vi "HFRR ADV v039.vi"() -> ()   [LabVIEW 2025] (continued)
                  tunnel: [w3880] -> w3851
                  n3077 = call-dynamic "Set Report Tab Width.vi"("report in"=w3883, "error in (no error)"=w3881) -> ("report out"=w3882:refnum<class "NI_report.lvclass">, "error out"=w3880:errorcluster)  [unwired: 12 in]
                }
                n3078 = control-ref of="Tab Control 9"() -> (w3847:refnum<vi>)
                n3079 = call-dynamic "Append Control Image to Report.vi"("report in"=w3852, "alignment (default)"=HTML_Report_Image_Alignment."ABSMIDDLE", "ctrl reference"=w3847, "error in (no error)"=w3851) -> ("report out"=w3846:refnum<class "NI_report.lvclass">, "error out"=w3845:errorcluster)  [unwired: 8 in, 2 out]
                n3080 = for {
                  N: 3 -> [_]
                  tunnel: [w3879] -> w3830
                  tunnel: [w3878] -> w3829
                  tunnel: w3846 -> [w3877]
                  tunnel: w3845 -> [w3876]
                  n3081 = call-dynamic "New Report Line.vi"("report in"=w3877, "error in (no error)"=w3876) -> ("report out"=w3879:refnum<class "NI_report.lvclass">, "error out"=w3878:errorcluster)  [unwired: 12 in]
                }
                n3082 = for {
                  N: 100 -> [_]
                  tunnel: w3830 -> [w3875]
                  tunnel: w3829 -> [w3873]
                  tunnel: [w3874] -> w3826
                  tunnel: [w3872] -> w3824
                  n3083 = call-dynamic "Set Report Tab Width.vi"("report in"=w3875, "error in (no error)"=w3873) -> ("report out"=w3874:refnum<class "NI_report.lvclass">, "error out"=w3872:errorcluster)  [unwired: 12 in]
                }
                n3084 = String To Path(string="C:\\LAB-IQ\\im\\Temp_resized.jpg") -> (path=w3816:path)
                n3085 = call-poly <vilib>:"Append Image to Report.vi"("report in"=w3826, "path or URL of image"=w3816, "error in (no error)"=w3824) -> ("report out"=w3825:refnum<class "NI_report.lvclass">, "error out"=w3823:errorcluster)  [unwired: 9 in, 2 out]
                n3086 = call-poly <vilib>:"Open HTML Report in Browser.vi"("report in"=w3825, "error in (no error)"=w3823) -> ("report out"=w3860:refnum<class "NI_report.lvclass">, "error out"=w3859:errorcluster)  [unwired: 11 in, 1 out]
                n3087 = call-dynamic "Dispose Report.vi"("report in"=w3860, "error in (no error)"=w3859) -> ()  [unwired: 13 in, 1 out]
              }
              frame #2 {
              }
              frame #3 {
                n3088 = disable-structure shown="Disabled" {
                  frame Disabled {
                    n3089 = local read "String 10"() -> (w3900:string)
                    n3090 = Concatenate Strings("C:\\LAB-IQ-NXT\\Data\\" ("string"), w3900, ".jpg" ("string")) -> (w3898:string)
                    n3091 = String To Path(string=w3898) -> (path=w3897:path)
                    n3092 = Delete(path (use dialog)=w3897) -> ()  [unwired: 4 in, 3 out]
                  }
                  frame Enabled {
                  }
                }
                n3093 = local write "Print 2"(FALSE ("Print")) -> ()
              }
            }
          }
        }
      }
    }
    n3094 = Wait (ms)(milliseconds to wait=u32 50) -> ()  [unwired: 1 out]
    n3095 = Wait (ms)(milliseconds to wait=u32 50) -> ()  [unwired: 1 out]
    n3096 = local read "Quit"() -> (w2242:bool)
  }
  n3097 = VISA Close(VISA resource name=w41, error in (no error)=w40) -> ()  [unwired: 1 out]
  n3098 = while {
    stop <- w4051 stop-if-true
    n3099 = local read "Auto Start Test"() -> (w4049:bool)
    n3100 = local read "RUN"() -> (w4048:bool)
    n3101 = Wait (ms)(milliseconds to wait=u32 1000) -> ()  [unwired: 1 out]
    n3102 = Or(x=w4048, y=w4049) -> (x .or. y?=w4047:bool)
    n3103 = case shown="True" w4047 {
      frame False {
      }
      frame True {
        n3104 = local read "LVDT STROKE Actual"() -> (w4052:dbl)
        n3105 = In Range and Coerce(upper limit=1.2, x=w4052, lower limit=0.6) -> (In Range?=w4055:bool)  [unwired: 1 out]
        n3106 = call-poly <vilib>:"Random Number (Range).vi"("lower bound (0)"=0.998 ("upper bound (100)"), "upper bound (100)"=1.003) -> ("number"=w4053:dbl)  [unwired: 9 in]
        n3107 = case shown="True" w4055 {
          tunnel: [w4060 w4061] -> w4054
          tunnel: w4053 -> [_ w4061]
          tunnel: w4052 -> [w4060 _]
          frame False {
          }
          frame True {
          }
        }
        "LVDT STROKE DISPLAY" <- w4054
      }
    }
    n3108 = local read "Quit"() -> (w4051:bool)
  }
  n3109 = while {
    tunnel: [w4078] -> w49
    shift-right: [w4071] -> _
    shift-left: 0.0 -> [w4074]
    shift-right: [w4070] -> _
    shift-left: 0.0 -> [w4073]
    shift-right: [w4069] -> _
    shift-left: 100.0 ("vc_cmd") -> [w4072]
    stop <- w4078 stop-if-true
    # "PID LOGIC"
    n3110 = local read "run test Calibration"() -> (w4066:bool)
    n3111 = local read "RUN"() -> (w4076:bool)
    n3112 = local read "Auto Start Temp"() -> (w4067:bool)
    n3113 = local read "Auto Start Test"() -> (w4075:bool)
    n3114 = local read "START TEMP"() -> (w4065:bool)
    n3115 = And(x=w4067, y=w4075) -> (x .and. y?=w4068:bool)
    n3116 = Or(x=w4076, y=w4068) -> (x .or. y?=w4077:bool)
    n3117 = And(x=w4077, y=w4065) -> (x .and. y?=w4064:bool)
    n3118 = And(x=w4066, y=w4065) -> (x .and. y?=w4063:bool)
    n3119 = Or(x=w4063, y=w4064) -> (x .or. y?=w4062:bool)
    n3120 = Wait (ms)(milliseconds to wait="milliseconds to wait") -> ()  [unwired: 1 out]
    n3121 = case shown="True" w4062 {
      tunnel: [400.0 ("out_vc_cmd") w4097] -> w4069
      tunnel: [w4081 w4099] -> w4070
      tunnel: [w4081 w4098] -> w4071
      tunnel: w4074 -> [_ w4088]
      tunnel: w4073 -> [_ w4087]
      tunnel: w4072 -> [_ w4086]
      tunnel: w4066 -> [_ w4082]
      frame False {
        w4081 = 0.0 ("error_out")
      }
      frame True {
        n3122 = case shown="True" w4082 {
          tunnel: [w4106 1.0] -> w4084
          frame False {
            n3123 = local read "Set Strk"() -> (w4105:dbl)
            n3124 = Add(x=w4105, y="Add up Stroke") -> (x+y=w4106:dbl)
          }
          frame True {
          }
        }
        n3125 = local read "LVDT STROKE"() -> (w4083:dbl)
        n3126 = formula code="// Zero-Hardcode Explicit Positional-Form PID Engine\n// Inputs: target_stroke, measured_stroke, dt, prev_error, integral_accumulator_in, prev_vc_cmd\n//         kp, ki, kd, max_step_change, max_amplitude, min_amplitude, startup_cmd\n// Outputs: vc_cmd, error_out, out_error, integral_accumulator_out, out_vc_cmd\n\n// 1. Calculate Tracking Error\nfloat current_error = target_stroke - measured_stroke;\nerror_out = current_error;\n\n// 2. Compute Proportional Term\nfloat p_term = kp * current_error;\n\n// 3. Compute Derivative Term\nfloat d_term = 0.0;\nif (dt > 0.0) {\n    d_term = kd * ((current_error - prev_error) / dt);\n}\n\n// 4. Update and Accumulate Integral Term\nfloat current_integral = integral_accumulator_in + (current_error * dt);\nfloat i_term = ki * current_integral;\n\n// 5. Calculate Ideal Target Command (Anchored by startup baseline)\nfloat ideal_command = startup_cmd + p_term + i_term + d_term;\n\n// 6. Apply Loop Rate Limiting FIRST \n// (Forces the command to climb gradually from prev_vc_cmd instead of jumping straight to max)\nfloat raw_adjustment = ideal_command - prev_vc_cmd;\n\nif (raw_adjustment > max_step_change) {\n    raw_adjustment = max_step_change;\n} else if (raw_adjustment < -max_step_change) {\n    raw_adjustment = -max_step_change;\n}\n\nfloat next_vc_cmd = prev_vc_cmd + raw_adjustment;\n\n// 7. Anti-Windup Protection & Final Output Safety Safeguard Clamping\n// (Back-calculating based on what we are ACTUALLY outputting)\nif (next_vc_cmd > max_amplitude) {\n    float excess = next_vc_cmd - max_amplitude;\n    if (ki > 0.0) {\n        current_integral -= excess / ki;\n    }\n    next_vc_cmd = max_amplitude;\n} else if (next_vc_cmd < min_amplitude) {\n    float excess = next_vc_cmd - min_amplitude;\n    if (ki > 0.0) {\n        current_integral -= excess / ki;\n    }\n    next_vc_cmd = min_amplitude;\n}\n\n// 8. Map to Shift Registers for memory persistence\nvc_cmd = next_vc_cmd;\nout_error = current_error;                   \nintegral_accumulator_out = current_integral;  \nout_vc_cmd = next_vc_cmd;"("target_stroke"=w4084, "measured_stroke"=w4083, "dt"="dt", "integral_accumulator_in"=w4087, "prev_error"=w4088, "prev_vc_cmd"=w4086, "kp"="kp", "ki"="ki", "kd"="kd", "max_step_change"="max_step_change", "max_amplitude"="max_amplitude", "min_amplitude"="min_amplitude", "startup_cmd"="startup_cmd") -> ("vc_cmd"=w4103:dbl, "out_error"=w4098:dbl, "integral_accumulator_out"=w4099:dbl, "out_vc_cmd"=w4097:dbl)  [unwired: 1 out]
        "output Vpp" <- w4103
        n3127 = Number To Fractional String(number=w4103, precision (6)=i16 1) -> (F-format string=w4101:string)  [unwired: 2 in]
        n3128 = Concatenate Strings("DAC;" ("string"), w4101) -> (w4085:string)
        n3129 = local write "Due Write"(w4085) -> ()
        "prev_error" <- w4088
        "integral_accumulator_in" <- w4087
        "prev_vc_cmd" <- w4086
      }
    }
    n3130 = local read "Quit"() -> (w4078:bool)
  }
  n3131 = Or(x=w45, y=w44) -> (x .or. y?=w46:bool)
  n3132 = Or(x=w42, y=w46) -> (x .or. y?=w51:bool)
  n3133 = control-ref of="new picture"() -> ()  [unwired: 1 out]
  n3134 = Or(x=w54, y=w51) -> (x .or. y?=w48:bool)
  n3135 = Or(x=w48, y=w49) -> (x .or. y?=w43:bool)
  n3136 = while {
    tunnel: [w4108] -> w53
    i -> [w4115]
    stop <- w4108 stop-if-true
    n3137 = local read "Quit"() -> (w4108:bool)
    n3138 = Equal To 0?(x=w4115) -> (x = 0?=w4113:bool)
    n3139 = call "Elapsed Time3"("Time Target (s)"=45.0, "Auto Reset"=TRUE) -> ("Time has Elapsed"=w4112:bool)  [unwired: 10 in, 7 out]
    n3140 = Wait (ms)(milliseconds to wait=u32 50) -> ()  [unwired: 1 out]
    n3141 = Or(x=w4112, y=w4113) -> (x .or. y?=w4114:bool)
    n3142 = case shown="True" w4114 {
      frame False {
      }
      frame True {
        n3143 = call <vilib>:"System Exec.vi"("run minimized? (F)"=TRUE, "error in (no error)"="error in (no error)", "command line"="powercfg.exe -change -monitor-timeout-ac 0") -> ("error out"=w4126:errorcluster)  [unwired: 5 in, 3 out]
        n3144 = call <vilib>:"System Exec.vi"("run minimized? (F)"=TRUE, "error in (no error)"=w4126, "command line"="powercfg.exe -change -disk-timeout-ac 0") -> ("error out"=w4125:errorcluster)  [unwired: 5 in, 3 out]
        n3145 = call <vilib>:"System Exec.vi"("run minimized? (F)"=TRUE, "error in (no error)"=w4125, "command line"="powercfg.exe -change -standby-timeout-ac 0") -> ("error out"=w4124:errorcluster)  [unwired: 5 in, 3 out]
        n3146 = call <vilib>:"System Exec.vi"("run minimized? (F)"=TRUE, "error in (no error)"=w4124, "command line"="powercfg.exe -change -hibernate-timeout-ac 0") -> ("error out"=w4123:errorcluster)  [unwired: 5 in, 3 out]
        n3147 = call <vilib>:"Simple Error Handler.vi"("error in (no error)"=w4123) -> ("error out"=w4129:errorcluster)  [unwired: 4 in, 4 out]
        n3148 = call <vilib>:"Clear Errors.vi"("error in (no error)"=w4129) -> ("error out"=→"error out":errorcluster)  [unwired: 5 in, 1 out]
      }
    }
  }
  n3149 = Compound Arithmetic op=OR(w56, w43, w53) -> (w55:bool)
  n3150 = flat-sequence {
    tunnel: w55 -> [_]
    tunnel: [w4131] -> w25
    tunnel: w25 -> [_]
    frame #0 {
      n3151 = call "CLOSE CONNECTION.vi"() -> ("error out"=w4131:errorcluster)  [unwired: 11 in]
    }
    frame #1 {
      n3152 = Quit LabVIEW(quit? (T)=TRUE) -> ()
      n3153 = local write "Quit"(FALSE ("EXIT")) -> ()
    }
  }
  n3154 = property on="Heater Button" class="Bool (strict)"("Visible"=TRUE) -> ()  [unwired: 2 in, 2 out]
  n3155 = while {
    tunnel: [w4138] -> _
    i -> [w4138]
    stop <- w4134 stop-if-true
    # "Langauage selection"
    n3156 = Equal?(x="Lan flag", y=22.0) -> ()  [unwired: 1 out]
    n3157 = disable-structure shown="Disabled" {
      frame Disabled {
        n3158 = stacked-sequence {
          frame #0 {
            n3159 = case shown="\"Russian\"" "Language Selection" {
              tunnel: [0 1] -> w4140
              frame "English", Default {
              }
              frame "Russian" {
              }
            }
            n3160 = for {
              N: 130 -> [_]
              tunnel: "Table" -> [w4149]
              tunnel: w4140 -> [w4148]
              i -> [w4147]
              n3161 = Index Array(array=w4149, index (row)=w4147, index (col)=w4148) -> (element=w4146:string)
              n3162 = case shown="1" w4147 {
                tunnel: w4146 -> [w4150 w4151 _ w4152 w4153 w4154 w4155 w4156 w4157 w4158 w4159 w4160 w4161 w4162 w4163 w4164 w4165 w4166 w4167 w4168 w4169 w4170 w4171 w4172 w4173 w4174 w4175 w4176 w4177 _ _ w4178 w4179 w4180 w4181 w4182 w4183 w4192 w4199 w4206 w4213 w4217 w4220 w4223 w4225 w4227 w4228 w4229 w4230 w4231 w4232 w4233 w4234 w4235 w4236 w4237 w4238 w4239 w4240 w4241 w4242 w4243 w4244 w4245 w4246 w4247 w4248 w4249 w4250 w4251 w4252 w4253 w4254 w4255 w4256 w4257 w4258 w4259 w4260 w4261 w4262 w4263 w4264 w4265 w4266 w4267 w4268 w4269 w4270 w4271 w4272 w4273 w4274 w4275 w4276 w4277 w4278 w4279 w4280 w4281 w4282 w4283 w4284 w4285 w4286 _ w4287 w4288 w4289 w4290 w4291 w4292 w4293 w4294 w4295 w4296 w4297 w4298 w4299 _ w4300 w4301 w4302 w4303 w4304 w4305 _]
                frame 0 {
                  n3163 = local write "S"(w4150) -> ()
                }
                frame 1 {
                  n3164 = local write "S 2"(w4151) -> ()
                }
                frame 2 {
                }
                frame 3 {
                  n3165 = local write "S 4"(w4152) -> ()
                }
                frame 4 {
                  n3166 = property on="FILE" class="Str"("Caption.Text"=w4153) -> ()  [unwired: 2 in, 2 out]
                }
                frame 5 {
                  n3167 = property on="Fuel Discription :" class="Str"("Caption.Text"=w4154) -> ()  [unwired: 2 in, 2 out]
                }
                frame 6 {
                  n3168 = property on="Remarks :" class="Str"("Caption.Text"=w4155) -> ()  [unwired: 2 in, 2 out]
                }
                frame 7 {
                  n3169 = property on="Save & Continue" class="Bool (strict)"("Boolean Text.Text"=w4156) -> ()  [unwired: 2 in, 2 out]
                }
                frame 8 {
                }
                frame 9 {
                  n3170 = property on="Set Hz" class="DigNum (strict)"("Caption.Text"=w4158) -> ()  [unwired: 2 in, 2 out]
                }
                frame 10 {
                }
                frame 11 {
                  n3171 = property on="NORMAL LOAD" class="DigNum (strict)"("Caption.Text"=w4160) -> ()  [unwired: 2 in, 2 out]
                }
                frame 12 {
                }
                frame 13 {
                  n3172 = property on="Set Temp" class="DigNum (strict)"("Caption.Text"=w4162) -> ()  [unwired: 2 in, 2 out]
                }
                frame 14 {
                  n3173 = local write "S 15"(w4163) -> ()
                }
                frame 15 {
                  n3174 = property on="Set Rh" class="DigNum (strict)"("Caption.Text"=w4164) -> ()  [unwired: 2 in, 2 out]
                }
                frame 16 {
                }
                frame 17 {
                  n3175 = local write "S 18"(w4166) -> ()
                }
                frame 18 {
                  "String 17" <- w4167
                }
                frame 19 {
                  n3176 = property on="test time" class="DigNum (strict)"("Caption.Text"=w4168) -> ()  [unwired: 2 in, 2 out]
                }
                frame 20 {
                  "String 18" <- w4169
                  "String 22" <- w4169
                }
                frame 21 {
                  n3177 = property on="Elapsed time" class="DigNum (strict)"("Caption.Text"=w4170) -> ()  [unwired: 2 in, 2 out]
                }
                frame 22 {
                  n3178 = property on="Samplingtime 2" class="DigNum (strict)"("Caption.Text"=w4171) -> ()  [unwired: 2 in, 2 out]
                }
                frame 23 {
                  "String 21" <- w4172
                }
                frame 24 {
                  n3179 = property on="Countdown" class="DigNum (strict)"("Caption.Text"=w4173) -> ()  [unwired: 2 in, 2 out]
                }
                frame 25 {
                  n3180 = property on="Countdown 2" class="DigNum (strict)"("Caption.Text"=w4174) -> ()  [unwired: 2 in, 2 out]
                }
                frame 26 {
                  n3181 = property on="Engage" class="Bool (strict)"("Boolean Text.Text"=w4175) -> ()  [unwired: 2 in, 2 out]
                }
                frame 27 {
                  n3182 = property on="Boolean  4" class="Bool (strict)"("Boolean Text.Text"=w4176) -> ()  [unwired: 2 in, 2 out]
                }
                frame 28 {
                  n3183 = property on="Test \nStatus" class="Bool (strict)"("Boolean Text.Text"=w4177) -> ()  [unwired: 2 in, 2 out]
                }
                frame 29 {
                }
                frame 30 {
                }
                frame 31 {
                }
                frame 32 {
                  n3184 = property on="RSTCOF" class="Bool"("Boolean Text.Text"=w4179) -> ()  [unwired: 2 in, 2 out]
                  n3185 = property on="RST FF" class="Bool"("Boolean Text.Text"=w4179) -> ()  [unwired: 2 in, 2 out]
                  n3186 = property on="RST TEMP" class="Bool"("Boolean Text.Text"=w4179) -> ()  [unwired: 2 in, 2 out]
                  n3187 = property on="RSTV1 3" class="Bool"("Boolean Text.Text"=w4179) -> ()  [unwired: 2 in, 2 out]
                  n3188 = property on="rstv2" class="Bool"("Boolean Text.Text"=w4179) -> ()  [unwired: 2 in, 2 out]
                  n3189 = property on="RSTV1 2" class="Bool"("Boolean Text.Text"=w4179) -> ()  [unwired: 2 in, 2 out]
                  n3190 = property on="RST CP" class="Bool"("Boolean Text.Text"=w4179) -> ()  [unwired: 2 in, 2 out]
                }
                frame 33 {
                  "S 61" <- w4180
                }
                frame 34 {
                  "String 23" <- w4181
                }
                frame 35 {
                  n3191 = property on="Rh Before" class="DigNum (strict)"("Caption.Text"=w4182) -> ()  [unwired: 2 in, 2 out]
                }
                frame 36 {
                  n3192 = Match Pattern(string=w4183, regular expression=",") -> (before substring=→"bs":string, after substring=→"as":string)  [unwired: 1 in, 2 out]
                  n3193 = property on="Rh After" class="DigNum (strict)"("Caption.Text"=w4183) -> ()  [unwired: 2 in, 2 out]
                }
                frame 37 {
                  n3194 = Match Pattern(string=w4192, regular expression=",") -> (before substring=w4191:string, after substring=w4190:string)  [unwired: 1 in, 2 out]
                  "bs" <- w4191
                  "as" <- w4190
                  n3195 = Concatenate Strings(w4191, w4190) -> (w4187:string)
                  n3196 = property on="Humidity before test 2" class="DigNum (strict)"("Caption.Text"=w4187) -> ()  [unwired: 2 in, 2 out]
                  n3197 = Concatenate Strings(w4187, "=" ("string")) -> (w4188:string)
                  n3198 = local write "S 38"(w4188) -> ()
                }
                frame 38 {
                  n3199 = Match Pattern(string=w4199, regular expression=",") -> (before substring=w4198:string, after substring=w4197:string)  [unwired: 1 in, 2 out]
                  "bs" <- w4198
                  "as" <- w4197
                  n3200 = Concatenate Strings(w4198, w4197) -> (w4194:string)
                  n3201 = property on="Humidity after test 2" class="DigNum (strict)"("Caption.Text"=w4194) -> ()  [unwired: 2 in, 2 out]
                  n3202 = Concatenate Strings(w4194, "=" ("string")) -> (w4196:string)
                  n3203 = local write "S 39"(w4196) -> ()
                }
                frame 39 {
                  n3204 = Match Pattern(string=w4206, regular expression=",") -> (before substring=w4205:string, after substring=w4204:string)  [unwired: 1 in, 2 out]
                  "bs" <- w4205
                  "as" <- w4204
                  n3205 = Concatenate Strings(w4205, w4204) -> (w4201:string)
                  n3206 = property on="Temperature before test 2" class="DigNum (strict)"("Caption.Text"=w4201) -> ()  [unwired: 2 in, 2 out]
                  n3207 = Concatenate Strings(w4201, "=" ("string")) -> (→"String 34":string)
                }
                frame 40 {
                  n3208 = Match Pattern(string=w4213, regular expression=",") -> (before substring=w4212:string, after substring=w4211:string)  [unwired: 1 in, 2 out]
                  "bs" <- w4212
                  "as" <- w4211
                  n3209 = Concatenate Strings(w4212, w4211) -> (w4208:string)
                  n3210 = property on="Temperature after test 2" class="DigNum (strict)"("Caption.Text"=w4208) -> ()  [unwired: 2 in, 2 out]
                  n3211 = Concatenate Strings(w4208, "=" ("string")) -> (→"String 35":string)
                  n3212 = property on="Temperature after test" class="DigNum (strict)"("Caption.Text"=w4208) -> ()  [unwired: 2 in, 2 out]
                }
                frame 41 {
                  n3213 = property on="AVP 2" class="DigNum (strict)"("Caption.Text"=w4217) -> ()  [unwired: 2 in, 2 out]
                  n3214 = Concatenate Strings(w4217, "=" ("string")) -> (→"String 36":string)
                }
                frame 42 {
                  n3215 = property on="MWSD 2" class="DigNum (strict)"("Caption.Text"=w4220) -> ()  [unwired: 2 in, 2 out]
                  n3216 = Concatenate Strings(w4220, "=" ("string")) -> (→"String 37":string)
                }
                frame 43 {
                  n3217 = property on="HCF 2" class="DigNum (strict)"("Caption.Text"=w4223) -> ()  [unwired: 2 in, 2 out]
                  n3218 = Concatenate Strings(w4223, "=" ("string")) -> (→"String 38":string)
                }
                frame 44 {
                  n3219 = Concatenate Strings(w4225, "=" ("string")) -> (→"String 39":string)
                  n3220 = property on="WS1.4 2" class="DigNum (strict)"("Caption.Text"=w4225) -> ()  [unwired: 2 in, 2 out]
                }
                frame 45 {
                }
                frame 46 {
                  n3221 = local write "S 47"(w4228) -> ()
                }
                frame 47 {
                  n3222 = local write "S 48"(w4229) -> ()
                }
                frame 48 {
                  n3223 = local write "S 49"(w4230) -> ()
                }
                frame 49 {
                  n3224 = local write "S 50"(w4231) -> ()
                }
                frame 50 {
                  n3225 = local write "S 51"(w4232) -> ()
                }
                frame 51 {
                  n3226 = local write "S 52"(w4233) -> ()
                }
                frame 52 {
                  n3227 = local write "S 53"(w4234) -> ()
                }
                frame 53 {
                  n3228 = local write "S 54"(w4235) -> ()
                }
                frame 54 {
                  n3229 = local write "S 55"(w4236) -> ()
                }
                frame 55 {
                  n3230 = local write "S 56"(w4237) -> ()
                }
                frame 56 {
                  n3231 = local write "S 57"(w4238) -> ()
                }
                frame 57 {
                  n3232 = local write "S 58"(w4239) -> ()
                }
                frame 58 {
                  n3233 = local write "S 59"(w4240) -> ()
                }
                frame 59 {
                  n3234 = local write "S 60"(w4241) -> ()
                }
                frame 60 {
                  n3235 = local write "S 62"(w4242) -> ()
                }
                frame 61 {
                  n3236 = local write "S 63"(w4243) -> ()
                }
                frame 62 {
                  n3237 = local write "S 64"(w4244) -> ()
                }
                frame 63 {
                  n3238 = local write "S 65"(w4245) -> ()
                }
                frame 64 {
                  n3239 = local write "S 66"(w4246) -> ()
                }
                frame 65 {
                  n3240 = local write "S 67"(w4247) -> ()
                }
                frame 66 {
                  n3241 = local write "S 68"(w4248) -> ()
                }
                frame 67 {
                  n3242 = local write "S 69"(w4249) -> ()
                }
                frame 68 {
                  n3243 = local write "S 70"(w4250) -> ()
                }
                frame 69 {
                  n3244 = local write "S 71"(w4251) -> ()
                }
                frame 70 {
                  n3245 = local write "S 72"(w4252) -> ()
                }
                frame 71 {
                  n3246 = local write "S 73"(w4253) -> ()
                }
                frame 72 {
                  n3247 = local write "S 74"(w4254) -> ()
                }
                frame 73 {
                  n3248 = local write "S 75"(w4255) -> ()
                }
                frame 74 {
                  n3249 = local write "S 76"(w4256) -> ()
                }
                frame 75 {
                  n3250 = local write "S 77"(w4257) -> ()
                }
                frame 76 {
                  n3251 = local write "S 78"(w4258) -> ()
                }
                frame 77 {
                  n3252 = local write "S 79"(w4259) -> ()
                }
                frame 79 {
                  n3253 = property on="Sample Temperature ( °C )" class="XYGraph (strict)"("Y Scale.Name Label.Text"=w4260) -> ()  [unwired: 2 in, 2 out]
                }
                frame 80 {
                  n3254 = local write "S 81"(w4261) -> ()
                  n3255 = property on="Humidity ( %RH )" class="XYGraph (strict)"("Y Scale.Name Label.Text"=w4261) -> ()  [unwired: 2 in, 2 out]
                }
                frame 78 {
                  n3256 = property on="Air Temperature  ( °C )" class="XYGraph (strict)"("X Scale.Name Label.Text"=w4262) -> ()  [unwired: 2 in, 2 out]
                  n3257 = property on="Humidity ( %RH )" class="XYGraph (strict)"("X Scale.Name Label.Text"=w4262) -> ()  [unwired: 2 in, 2 out]
                  n3258 = property on="Sample Temperature ( °C )" class="XYGraph (strict)"("X Scale.Name Label.Text"=w4262) -> ()  [unwired: 2 in, 2 out]
                  n3259 = property on="Coefficient Of Friction" class="XYGraph (strict)"("X Scale.Name Label.Text"=w4262) -> ()  [unwired: 2 in, 2 out]
                }
                frame 81 {
                  n3260 = property on="Air Temperature  ( °C )" class="XYGraph (strict)"("Y Scale.Name Label.Text"=w4263) -> ()  [unwired: 2 in, 2 out]
                }
                frame 82 {
                  n3261 = local write "S 84"(w4264) -> ()
                }
                frame 83 {
                  n3262 = local write "S 85"(w4265) -> ()
                }
                frame 84 {
                  n3263 = local write "S 86"(w4266) -> ()
                }
                frame 85 {
                  n3264 = local write "S 87"(w4267) -> ()
                }
                frame 86 {
                  n3265 = local write "S 88"(w4268) -> ()
                }
                frame 87 {
                }
                frame 88 {
                  n3266 = local write "S 90"(w4270) -> ()
                }
                frame 89 {
                  n3267 = local write "S 91"(w4271) -> ()
                }
                frame 90 {
                  n3268 = local write "S 92"(w4272) -> ()
                }
                frame 91 {
                  n3269 = local write "S 93"(w4273) -> ()
                }
                frame 92 {
                  n3270 = local write "S 94"(w4274) -> ()
                }
                frame 93 {
                  n3271 = local write "S 95"(w4275) -> ()
                }
                frame 94 {
                  n3272 = local write "S 96"(w4276) -> ()
                }
                frame 95 {
                  n3273 = local write "S 97"(w4277) -> ()
                }
                frame 96 {
                  n3274 = local write "S 98"(w4278) -> ()
                }
                frame 97 {
                  n3275 = local write "S 99"(w4279) -> ()
                }
                frame 98 {
                  n3276 = local write "S 100"(w4280) -> ()
                }
                frame 99 {
                  n3277 = local write "S 101"(w4281) -> ()
                }
                frame 100 {
                  n3278 = local write "S 102"(w4282) -> ()
                }
                frame 101 {
                  n3279 = local write "S 103"(w4283) -> ()
                }
                frame 102 {
                  n3280 = local write "S 104"(w4284) -> ()
                }
                frame 103 {
                  n3281 = local write "S 105"(w4285) -> ()
                }
                frame 104 {
                  n3282 = local write "S 106"(w4286) -> ()
                }
                frame 105 {
                }
                frame 106 {
                  n3283 = property on="OK Button 17" class="Bool (strict)"("Boolean Text.Text"=w4287) -> ()  [unwired: 2 in, 2 out]
                }
                frame 107 {
                  n3284 = property on="OK Button 16" class="Bool (strict)"("Boolean Text.Text"=w4288) -> ()  [unwired: 2 in, 2 out]
                }
                frame 108 {
                  n3285 = property on="TITTLE" class="Str"("Caption.Text"=w4289) -> ()  [unwired: 2 in, 2 out]
                }
                frame 109 {
                  "String 30" <- w4290
                }
                frame 110 {
                  n3286 = property on="Test Date" class="Str"("Caption.Text"=w4291) -> ()  [unwired: 2 in, 2 out]
                  "String 31" <- w4291
                }
                frame 111 {
                  n3287 = property on="Sample ID" class="Str"("Caption.Text"=w4292) -> ()  [unwired: 2 in, 2 out]
                  "String 32" <- w4292
                }
                frame 112 {
                  n3288 = property on="Tested by" class="Str"("Caption.Text"=w4293) -> ()  [unwired: 2 in, 2 out]
                  "String 33" <- w4293
                }
                frame 113 {
                  n3289 = property on="System Configured Printers 2" class="Arr (strict)"("Caption.Text"=w4294) -> ()  [unwired: 2 in, 2 out]
                }
                frame 114 {
                  n3290 = property on="Selected Printer" class="Str"("Caption.Text"=w4295) -> ()  [unwired: 2 in, 2 out]
                }
                frame 115 {
                  n3291 = property on="Select Printer 3" class="DigNum (strict)"("Caption.Text"=w4296) -> ()  [unwired: 2 in, 2 out]
                }
                frame 116 {
                  n3292 = property on="Print" class="Bool (strict)"("Boolean Text.Text"=w4297) -> ()  [unwired: 2 in, 2 out]
                }
                frame 117 {
                  "String 41" <- w4298
                }
                frame 118 {
                  n3293 = property on="tested by" class="Str"("Caption.Text"=w4299) -> ()  [unwired: 2 in, 2 out]
                }
                frame 119 {
                }
                frame 120 {
                  n3294 = property on="Export" class="Bool (strict)"("Boolean Text.Text"=w4300) -> ()  [unwired: 2 in, 2 out]
                }
                frame 121 {
                }
                frame 122 {
                }
                frame 123 {
                  n3295 = property on="Select File Type" class="Enum (strict)"("Caption.Text"=w4303) -> ()  [unwired: 2 in, 2 out]
                }
                frame 124 {
                  n3296 = property on="s.NO" class="Str"("Caption.Text"=w4304) -> ()  [unwired: 2 in, 2 out]
                  "String 45" <- w4304
                }
                frame 125 {
                  n3297 = property on="trip1 8" class="Bool (strict)"("Boolean Text.Text"=w4305) -> ()  [unwired: 2 in, 2 out]
                }
                frame 126, Default {
                }
              }
            }
          }
          frame #1 {
            w4313 = TRUE ("Visible")
            n3298 = local read "S 91"() -> (w4330:string)
            n3299 = local read "S 90"() -> (w4329:string)
            n3300 = local read "S 88"() -> (w4328:string)
            n3301 = property on="File Path" class="Path"("Caption.Text"=w4329) -> ()  [unwired: 2 in, 2 out]
            n3302 = local read "S 71"() -> (w4323:string)
            n3303 = local read "S 86"() -> (w4325:string)
            n3304 = local read "S 85"() -> (w4326:string)
            n3305 = local read "S 87"() -> (w4324:string)
            n3306 = local read "S 84"() -> (w4327:string)
            n3307 = local read "S 103"() -> (w4312:string)
            n3308 = local read "S 104"() -> (w4311:string)
            n3309 = property on="Password" class="Str"("Caption.Text"=w4326) -> ()  [unwired: 2 in, 2 out]
            n3310 = property on="EDIT" class="Bool (strict)"("Boolean Text.Text"=w4323) -> ()  [unwired: 2 in, 2 out]
            n3311 = property on="SAVE" class="Bool (strict)"("Boolean Text.Text"=w4327) -> ()  [unwired: 2 in, 2 out]
            n3312 = Build Array(w4312, w4311) -> (w4310:string[])
            n3313 = property on="Heater Button" class="Bool (strict)"("Strings [4]"=w4310) -> ()  [unwired: 2 in, 2 out]
            n3314 = local read "S 92"() -> (w4322:string)
            n3315 = local read "S 93"() -> (w4321:string)
            n3316 = local read "S 105"() -> (w4308:string)
            n3317 = local read "S 106"() -> (w4307:string)
            n3318 = Build Array(w4322, w4321) -> ()  [unwired: 1 out]
            n3319 = Build Array(w4308, w4307) -> (w4309:string[])
            n3320 = local read "S 95"() -> (w4319:string)
            n3321 = local read "S 94"() -> (w4320:string)
            n3322 = local read "bs"() -> (w4335:string)
            n3323 = local read "as"() -> (w4336:string)
            n3324 = property on="Humidity" class="Bool (strict)"("Strings [4]"=w4309) -> ()  [unwired: 2 in, 2 out]
            n3325 = Concatenate Strings(w4335, "\r", w4336) -> ()  [unwired: 1 out]
            n3326 = property on="Rh After" class="DigNum (strict)"("Caption.Size to Text?"=TRUE ("Caption.Size to Text")) -> ()  [unwired: 2 in, 2 out]
            n3327 = local read "S 48"() -> (w4359:string)
            n3328 = local read "S 50"() -> (w4357:string)
            n3329 = local read "S 51"() -> (w4356:string)
            n3330 = local read "S 49"() -> (w4358:string)
            n3331 = local read "S 52"() -> (w4355:string)
            n3332 = local read "as"() -> (w4340:string)
            n3333 = local read "bs"() -> (w4341:string)
            n3334 = local read "S 56"() -> (w4354:string)
            n3335 = local read "S 57"() -> (w4353:string)
            n3336 = local read "S 58"() -> (w4352:string)
            n3337 = local read "S 59"() -> (w4351:string)
            n3338 = property on="OPEN" class="Bool (strict)"("Boolean Text.Text"=w4355) -> ()  [unwired: 2 in, 2 out]
            n3339 = property on="OPEN 1" class="Bool (strict)"("Boolean Text.Text"=w4359) -> ()  [unwired: 2 in, 2 out]
            n3340 = property on="OPEN 2" class="Bool (strict)"("Boolean Text.Text"=w4358) -> ()  [unwired: 2 in, 2 out]
            n3341 = property on="OPEN 3" class="Bool (strict)"("Boolean Text.Text"=w4357) -> ()  [unwired: 2 in, 2 out]
            n3342 = property on="OPEN 4" class="Bool (strict)"("Boolean Text.Text"=w4356) -> ()  [unwired: 2 in, 2 out]
            n3343 = Concatenate Strings(w4341, "\r", w4340) -> ()  [unwired: 1 out]
            n3344 = local read "S 102"() -> (w4314:string)
            n3345 = property on="КОФ1" class="DigNum (strict)"("Caption.Text"=w4354) -> ()  [unwired: 2 in, 2 out]
            n3346 = local read "S 98"() -> (w4318:string)
            n3347 = local read "S 99"() -> (w4317:string)
            n3348 = local read "S 100"() -> (w4316:string)
            n3349 = local read "S 101"() -> (w4315:string)
            n3350 = property on="КОФ2" class="DigNum (strict)"("Caption.Text"=w4353) -> ()  [unwired: 2 in, 2 out]
            n3351 = property on="КОФ3" class="DigNum (strict)"("Caption.Text"=w4352) -> ()  [unwired: 2 in, 2 out]
            n3352 = property on="КОФ4" class="DigNum (strict)"("Caption.Text"=w4351) -> ()  [unwired: 2 in, 2 out]
            n3353 = local read "bs"() -> (w4339:string)
            n3354 = local read "as"() -> (w4338:string)
            n3355 = local read "S 60"() -> (w4350:string)
            n3356 = local read "S 54"() -> (w4360:string)
            n3357 = Concatenate Strings(w4339, "\r", w4338) -> ()  [unwired: 1 out]
            n3358 = Concatenate Strings(w4360, w4350) -> ()  [unwired: 1 out]
            n3359 = local read "S 77"() -> (→"String 43":string)
            n3360 = local read "S 76"() -> (w4333:string)
            n3361 = local read "S 78"() -> (w4332:string)
            n3362 = local read "S 71"() -> (w4344:string)
            n3363 = local read "S 66"() -> (w4349:string)
            n3364 = local read "S 67"() -> (w4348:string)
            n3365 = local read "S 68"() -> (w4347:string)
            n3366 = local read "S 69"() -> (w4346:string)
            n3367 = local read "S 70"() -> (w4345:string)
            n3368 = property on="AIR TEMP" class="DigNum (strict)"("Caption.Text"=w4332) -> ()  [unwired: 2 in, 2 out]
            n3369 = property on="Set Strk" class="DigNum (strict)"("Caption.Text"=w4333) -> ()  [unwired: 2 in, 2 out]
            n3370 = property on="SPEED OUT:" class="DigNum (strict)"("Caption.Text"=w4347) -> ()  [unwired: 2 in, 2 out]
            n3371 = property on="EDIT" class="Bool (strict)"("Boolean Text.Text"=w4344) -> ()  [unwired: 2 in, 2 out]
            n3372 = local read "S 79"() -> (w4331:string)
          }
          frame #2 {
          }
        }
        n3373 = local write "Lan flag"(10.0 ("Lan flag")) -> ()
      }
      frame Enabled {
      }
    }
    n3374 = Wait (ms)(milliseconds to wait=u32 2000) -> ()  [unwired: 1 out]
    n3375 = local read "Quit"() -> (w4134:bool)
  }
  n3376 = while {
    shift-right: [w4366] -> _
    shift-left: _ -> [w4367]
    shift-right: [w4364] -> _
    shift-left: T18 {"Read Heave and Surge"="", "Bytes at Heave Port"=0.0, "Heave and Surge COM Port:"="COM9", "Com Port 2"="COM7", "Residual Due"="", "Heave COM Status 2"=TRUE, "Heave COM Status"=TRUE, "Port 2"=TRUE, "Sway PPR"=6400.0, "Surge PPR"=6400.0, "Heave PPR"=6400.0, "Sway Pitch"=2.0, "Surge Pitch"=3.0, "Heave Pitch"=4.0, "Sway Pulses/mm"=320.0, "Surge Pulses/mm"=1600.0, "Heave Pulses/mm"=1600.0, "inner loop"=0.0, "Read Heave and Surge 2"="", "String 36"="", "Write S"=FALSE, "WriteCC1"=[""], "Heave COM Loop"=0, "LastCom"="", "EXIT"=FALSE, "Error Heave"={"status"=TRUE, "code"=-1073807343, "source"=""}} -> [w4363]
    shift-right: [w4361] -> _
    shift-left: enum16{"init", "MAIN", "Panel Close"}."init" -> [w4362]
    stop <- w4365 stop-if-true
    # "HUMIDITY LOOP LOGIC"
    n3377 = case shown="\"MAIN\"" w4362 {
      tunnel: w4367 -> [w4381 w4405 w4469 w4471]
      tunnel: [w4376 w4392 w4469 w4471] -> w4366
      tunnel: [_ _ TRUE _] -> w4365
      tunnel: [w4373 w4390 w4467 w4470] -> w4364
      tunnel: w4363 -> [w4378 w4404 w4467 w4470]
      tunnel: [enum16{"init", "MAIN", "Panel Close"}."MAIN" w4399 _ _] -> w4361
      frame "init" {
        n3378 = local read "C3 :"() -> (w4368:refnum<visa-resource-name>)
        n3379 = Bundle By Name(cluster=w4378, "Heave and Surge COM Port:"=w4368) -> (w4377:T18)
        n3380 = call "Instrument fgv uno.vi"("Enum"=T32."INIT", "error in (no error) 2"=w4381, "INPUT"=w4377) -> ("error"=w4379:errorcluster, "output"=w4375:T18)  [unwired: 6 in, 1 out]
        n3381 = case shown="Error" w4379 {
          selector: w4379 -> [w4383 _]
          tunnel: [w4383 w4387] -> w4376
          tunnel: w4375 -> [w4382 w4385]
          tunnel: [w4382 w4384] -> w4374
          frame No Error {
          }
          frame Error {
            n3382 = call "Instrument fgv uno.vi"("Enum"=T32."ERROR INIT", "INPUT"=w4385) -> ("error"=w4388:errorcluster, "output"=w4384:T18)  [unwired: 7 in, 1 out]
            n3383 = call <vilib>:"Clear Errors.vi"("error in (no error)"=w4388) -> ("error out"=w4387:errorcluster)  [unwired: 5 in, 1 out]
          }
        }
        n3384 = local read "LastCom Humidity"() -> (w4371:string)
        n3385 = Unbundle By Name(w4374) -> ("Heave COM Status 2"=→"COM Status":bool, "Error Heave"=→"Error":errorcluster)  [unwired: 1 out]
        n3386 = Bundle By Name(cluster=w4374, "LastCom"=w4371) -> (w4373:T18)
      }
      frame "MAIN" {
        n3387 = Unbundle By Name(w4404) -> ("Com Port 2"=w4394:refnum<visa-resource-name>)
        n3388 = local read "C3 :"() -> (w4395:refnum<visa-resource-name>)
        n3389 = local write "COM Port Humidity :"(w4394) -> ()
        n3390 = Bundle By Name(cluster=w4404, "Heave and Surge COM Port:"=w4395) -> (w4403:T18)
        n3391 = Equal?(x=w4394, y=w4395) -> (x = y?=w4408:bool)
        n3392 = case shown="True" w4408 {
          tunnel: [w4423 w4440] -> w4393
          tunnel: w4405 -> [w4424 w4446]
          tunnel: w4403 -> [w4422 w4444]
          tunnel: [w4421 w4439] -> w4391
          frame False {
            n3393 = call <vilib>:"Clear Errors.vi"("error in (no error)"=w4424) -> ("error out"=w4420:errorcluster)  [unwired: 5 in, 1 out]
            n3394 = call "Instrument fgv uno.vi"("Enum"=T32."ERROR INIT", "error in (no error) 2"=w4420, "INPUT"=w4422) -> ("error"=w4426:errorcluster, "output"=w4421:T18)  [unwired: 6 in, 1 out]
            n3395 = call <vilib>:"Clear Errors.vi"("error in (no error)"=w4426) -> ("error out"=w4423:errorcluster)  [unwired: 5 in, 1 out]
          }
          frame True {
            n3396 = call "Instrument fgv uno.vi"("Enum"=T32."READ", "error in (no error) 2"=w4446, "INPUT"=w4444) -> ("error"=w4445:errorcluster, "output"=w4438:T18)  [unwired: 6 in, 1 out]
            n3397 = Bundle By Name(cluster=w4438, "String 36"="WRITE HUMIDITY") -> (w4437:T18)
            n3398 = case shown="True" "Write Humidity" {
              selector: "Write Humidity" -> [_ w4466]
              tunnel: w4445 -> [w4459 w4465]
              tunnel: [w4459 w4464] -> w4435
              tunnel: w4437 -> [w4458 w4462]
              tunnel: [w4458 w4461] -> w4434
              frame False {
              }
              frame True {
                n3399 = Not(x=w4466) -> (.not. x?=w4460:bool)
                n3400 = local write "Write Humidity"(w4460) -> ()
                n3401 = call "Instrument fgv uno.vi"("Enum"=T32."MANUAL WRITE", "error in (no error) 2"=w4465, "INPUT"=w4462) -> ("error"=w4464:errorcluster, "output"=w4461:T18)  [unwired: 6 in, 1 out]
              }
            }
            n3402 = Array Size(array="WriteHumidity") -> (size(s)=w4432:i32)
            n3403 = Greater Than 0?(x=w4432) -> (x > 0?=w4431:bool)
            n3404 = call "Instrument fgv uno.vi"("Enum"=T32."WRITE", "error in (no error) 2"=w4435, "WriteCC1"="WriteHumidity", "INPUT"=w4434) -> ("error"=w4442:errorcluster, "WriteCC1 2"=w4433:string[], "output"=w4441:T18)  [unwired: 5 in]
            n3405 = case shown="True" w4431 {
              tunnel: w4433 -> [_ w4448]
              frame False {
              }
              frame True {
                n3406 = local write "WriteHumidity"(w4448) -> ()
              }
            }
            n3407 = case shown="No Error" w4442 {
              selector: w4442 -> [w4449 w4452]
              tunnel: w4441 -> [w4450 w4457]
              tunnel: [w4450 w4456] -> w4439
              tunnel: [w4449 w4454] -> w4440
              frame No Error {
              }
              frame Error {
                n3408 = call <vilib>:"Clear Errors.vi"("error in (no error)"=w4452) -> ("error out"=w4451:errorcluster)  [unwired: 5 in, 1 out]
                n3409 = call "Instrument fgv uno.vi"("Enum"=T32."ERROR INIT", "error in (no error) 2"=w4451, "INPUT"=w4457) -> ("error"=w4455:errorcluster, "output"=w4456:T18)  [unwired: 6 in, 1 out]
                n3410 = call <vilib>:"Clear Errors.vi"("error in (no error)"=w4455) -> ("error out"=w4454:errorcluster)  [unwired: 5 in, 1 out]
              }
            }
            n3411 = Unbundle By Name(w4439) -> ("LastCom"=→"LastCom Humidity":string, "Read Heave and Surge"=→"Read HUMIDITY":string)
          }
        }
        n3412 = Unbundle By Name(w4391) -> ("Heave COM Status 2"=w4407:bool, "Error Heave"=w4396:errorcluster, "Bytes at Heave Port"=→"Bytes at Humidity Port  2":dbl)  [unwired: 1 out]
        n3413 = Unbundle By Name(w4396) -> ("status"=→"Humidity Port":bool)
        n3414 = Not(x=w4407) -> (.not. x?=w4397:bool)
        n3415 = local write "Error"(w4396) -> ()
        n3416 = local read "Quit"() -> (w4400:bool)
        n3417 = local write "COM Status"(w4397) -> ()
        n3418 = Select(t=enum16{"init", "MAIN", "Panel Close"}."Panel Close", s=w4400, f=enum16{"init", "MAIN", "Panel Close"}."MAIN") -> (s? t:f=w4399:enum16{"init", "MAIN", "Panel Close"})
        n3419 = local read "Humidity 2"() -> (w4389:bool)
        n3420 = case shown="True" w4389 {
          selector: w4389 -> [_ w4411]
          tunnel: w4393 -> [w4409 w4416]
          tunnel: [w4409 w4415] -> w4392
          tunnel: w4391 -> [w4410 w4414]
          tunnel: [w4410 w4413] -> w4390
          frame False {
          }
          frame True {
            n3421 = Not(x=w4411) -> (.not. x?=→"Humidity 2":bool)
            n3422 = call <vilib>:"Clear Errors.vi"("error in (no error)"=w4416) -> ("error out"=w4419:errorcluster)  [unwired: 5 in, 1 out]
            n3423 = call "Instrument fgv uno.vi"("Enum"=T32."ERROR INIT", "error in (no error) 2"=w4419, "INPUT"=w4414) -> ("error"=w4417:errorcluster, "output"=w4413:T18)  [unwired: 6 in, 1 out]
            n3424 = call <vilib>:"Clear Errors.vi"("error in (no error)"=w4417) -> ("error out"=w4415:errorcluster)  [unwired: 5 in, 1 out]
          }
        }
      }
      frame "Panel Close" {
      }
      frame Default {
      }
    }
  }
  n3425 = while {
    stop <- w4473 stop-if-true
    n3426 = call <vilib>:"High Resolution Polling Wait.vi"("seconds to wait"=0.05) -> ()  [unwired: 10 in, 1 out]
    n3427 = disable-structure shown="Enabled" {
      frame Disabled {
        n3428 = local read "Read HUMIDITY"() -> (w4474:string)
        n3429 = Spreadsheet String To Array(delimiter (Tab)=",", format string="", spreadsheet string=w4474, array type (2D Dbl)=string[] []) -> (array=w4493:string[])
        n3430 = for {
          tunnel: w4493 -> [w4502] mode=indexing
          tunnel: string[] ["STATE;", "SET;", "RH;", "T;", "AMB_RH;", "AMB_T;", "PUMP;", "FAN_IN;", "FAN_OUT;", "DEHUM;", "CURRENT;", "STALL;"] -> [w4501] mode=indexing
          tunnel: [w4500] -> w4492 mode=indexing
          n3431 = Match Pattern(string=w4502, regular expression=w4501) -> (after substring=w4500:string)  [unwired: 1 in, 3 out]
        }
        n3432 = Index Array(array=w4492) -> (element #1=w4491:string, element #2=w4490:string, element #3=w4482:string, element #4=w4481:string, element #5=w4480:string, element #6=w4489:string, element #7=w4488:string, element #8=w4487:string, element #9=w4486:string, element #10=w4485:string, element #11=w4484:string, element #12=w4483:string)  [unwired: 12 in]
        n3433 = Fract/Exp String To Number(string=w4482) -> (number=w4475:dbl)  [unwired: 3 in, 1 out]
        n3434 = Fract/Exp String To Number(string=w4480) -> (number=w4479:dbl)  [unwired: 3 in, 1 out]
        n3435 = local write "Ambient Humidity :"(w4479) -> ()
        n3436 = Equal?(x=w4475, y=0.0) -> (x = y?=w4477:bool)
        n3437 = case shown="True" w4477 {
          tunnel: [w4498 w4499] -> w4476
          tunnel: w4475 -> [w4498 _]
          frame False {
            (unwired) 0.0
            "Humidity temp" <- w4498
          }
          frame True {
            n3438 = local read "Humidity temp"() -> (w4499:dbl)
          }
        }
        "RH Numeric:" <- w4476
      }
      frame Enabled {
        n3439 = local read "Read HUMIDITY"() -> (w4522:string)
        n3440 = Spreadsheet String To Array(delimiter (Tab)=",", format string="", spreadsheet string=w4522, array type (2D Dbl)=dbl[] []) -> (array=w4518:dbl[])
        n3441 = Index Array(array=w4518) -> (element #1=→"STATE :":dbl, element #2=→"SET :":dbl, element #3=w4503:dbl, element #4=→"T :":dbl, element #5=→"AMB_RH :":dbl, element #6=→"AMB_T :":dbl, element #7=→"PUMP :":dbl, element #8=→"FAN_IN :":dbl, element #9=→"FAN_OUT :":dbl, element #10=→"DEHUM :":dbl, element #11=→"CURRENT :":dbl, element #12=→"STALL":dbl)  [unwired: 12 in]
        "RH :" <- w4503
        n3442 = Equal?(x=w4503, y=0.0) -> (x = y?=w4506:bool)
        n3443 = case shown="False" w4506 {
          tunnel: [w4523 w4524] -> w4507
          tunnel: w4503 -> [w4523 _]
          frame False {
            "Humidity temp 2" <- w4523
          }
          frame True {
            n3444 = local read "Humidity temp 2"() -> (w4524:dbl)
          }
        }
        n3445 = local write "RH Numeric:"(w4507) -> ()
      }
    }
    n3446 = local read "Quit"() -> (w4473:bool)
  }
  n3447 = while {
    shift-right: [w4530] -> _
    shift-left: _ -> [w4531]
    shift-right: [w4528] -> _
    shift-left: T20 {"Read Uno"="", "Bytes at Heave Port"=0.0, "UNO COM Port:"="COM9", "UNO COM Port: 2"="COM7", "Residual Due"="", "UNO COM Status 2"=TRUE, "UNO COM Status"=TRUE, "Port 2"=TRUE, "Sway PPR"=6400.0, "Surge PPR"=6400.0, "Heave PPR"=6400.0, "Sway Pitch"=2.0, "Surge Pitch"=3.0, "Heave Pitch"=4.0, "Sway Pulses/mm"=320.0, "Surge Pulses/mm"=1600.0, "Heave Pulses/mm"=1600.0, "inner loop"=0.0, "Read Heave and Surge 2"="", "String 36"="", "Write S"=FALSE, "WriteCC1"=[""], "Heave COM Loop"=0, "LastCom"="", "EXIT"=FALSE, "Error Heave"={"status"=TRUE, "code"=-1073807343, "source"=""}} -> [w4527]
    shift-right: [w4525] -> _
    shift-left: enum16{"init", "MAIN", "Panel Close"}."init" -> [w4526]
    stop <- w4529 stop-if-true
    # "UNO CODE LOGIC"
    n3448 = case shown="\"MAIN\"" w4526 {
      tunnel: w4531 -> [w4545 w4564 w4620 w4622]
      tunnel: [w4540 w4569 w4620 w4622] -> w4530
      tunnel: [_ _ TRUE _] -> w4529
      tunnel: [w4536 w4567 w4618 w4621] -> w4528
      tunnel: w4527 -> [w4542 w4563 w4618 w4621]
      tunnel: [enum16{"init", "MAIN", "Panel Close"}."MAIN" w4558 _ _] -> w4525
      frame "init" {
        n3449 = local read "Com Port 1"() -> (w4532:refnum<visa-resource-name>)
        n3450 = Bundle By Name(cluster=w4542, "UNO COM Port:"=w4532) -> (w4541:T20)
        n3451 = call "Instrument fgv.vi"("Enum"=T32."INIT", "error in (no error) 2"=w4545, "INPUT"=w4541) -> ("error"=w4543:errorcluster, "output"=w4539:T18)  [unwired: 6 in, 1 out]
        n3452 = case shown="Error" w4543 {
          selector: w4543 -> [w4547 _]
          tunnel: [w4547 w4551] -> w4540
          tunnel: w4539 -> [w4546 w4549]
          tunnel: [w4546 w4548] -> w4537
          frame No Error {
          }
          frame Error {
            n3453 = call "Instrument fgv.vi"("Enum"=T32."ERROR INIT", "INPUT"=w4549) -> ("error"=w4552:errorcluster, "output"=w4548:T18)  [unwired: 7 in, 1 out]
            n3454 = call <vilib>:"Clear Errors.vi"("error in (no error)"=w4552) -> ("error out"=w4551:errorcluster)  [unwired: 5 in, 1 out]
          }
        }
        n3455 = local read "LastCom UNO"() -> (w4534:string)
        n3456 = Unbundle By Name(w4537) -> ("Heave COM Status 2"=→"Instrument Status":bool, "Error Heave"=→"Error  2":errorcluster)  [unwired: 1 out]
        n3457 = Bundle By Name(cluster=w4537, "LastCom"=w4534) -> (w4536:T18)
      }
      frame "MAIN" {
        n3458 = Unbundle By Name(w4563) -> ("UNO COM Port: 2"=w4553:refnum<visa-resource-name>)
        n3459 = local read "Com Port 1"() -> (w4554:refnum<visa-resource-name>)
        n3460 = local write "COM Port UNO :"(w4553) -> ()
        n3461 = Equal?(x=w4553, y=w4554) -> (x = y?=w4570:bool)
        n3462 = Bundle By Name(cluster=w4563, "UNO COM Port:"=w4554) -> (w4562:T20)
        n3463 = case shown="True" w4570 {
          tunnel: [w4574 w4591] -> w4569
          tunnel: w4564 -> [w4575 w4597]
          tunnel: w4562 -> [w4573 w4595]
          tunnel: [w4572 w4590] -> w4567
          frame False {
            n3464 = call <vilib>:"Clear Errors.vi"("error in (no error)"=w4575) -> ("error out"=w4571:errorcluster)  [unwired: 5 in, 1 out]
            n3465 = call "Instrument fgv.vi"("Enum"=T32."ERROR INIT", "error in (no error) 2"=w4571, "INPUT"=w4573) -> ("error"=w4577:errorcluster, "output"=w4572:T18)  [unwired: 6 in, 1 out]
            n3466 = call <vilib>:"Clear Errors.vi"("error in (no error)"=w4577) -> ("error out"=w4574:errorcluster)  [unwired: 5 in, 1 out]
          }
          frame True {
            n3467 = call "Instrument fgv.vi"("Enum"=T32."READ", "error in (no error) 2"=w4597, "INPUT"=w4595) -> ("error"=w4596:errorcluster, "output"=w4589:T18)  [unwired: 6 in, 1 out]
            n3468 = Bundle By Name(cluster=w4589, "String 36"="WRITE UNO") -> (w4588:T18)
            n3469 = case shown="True" "Write" {
              selector: "Write" -> [_ w4612]
              tunnel: w4596 -> [w4610 w4617]
              tunnel: [w4610 w4616] -> w4586
              tunnel: w4588 -> [w4609 w4614]
              tunnel: [w4609 w4613] -> w4585
              frame False {
              }
              frame True {
                n3470 = Not(x=w4612) -> (.not. x?=w4611:bool)
                n3471 = local write "Write"(w4611) -> ()
                n3472 = call "Instrument fgv.vi"("Enum"=T32."MANUAL WRITE", "error in (no error) 2"=w4617, "INPUT"=w4614) -> ("error"=w4616:errorcluster, "output"=w4613:T18)  [unwired: 6 in, 1 out]
              }
            }
            n3473 = Array Size(array="Write UNO") -> (size(s)=w4583:i32)
            n3474 = Greater Than 0?(x=w4583) -> (x > 0?=w4582:bool)
            n3475 = call "Instrument fgv.vi"("Enum"=T32."WRITE", "error in (no error) 2"=w4586, "WriteCC1"="Write UNO", "INPUT"=w4585) -> ("error"=w4593:errorcluster, "WriteCC1 2"=w4584:string[], "output"=w4592:T18)  [unwired: 5 in]
            n3476 = case shown="True" w4582 {
              tunnel: w4584 -> [_ w4599]
              frame False {
              }
              frame True {
                n3477 = local write "Write UNO"(w4599) -> ()
              }
            }
            n3478 = case shown="Error" w4593 {
              selector: w4593 -> [w4600 w4603]
              tunnel: w4592 -> [w4601 w4608]
              tunnel: [w4601 w4607] -> w4590
              tunnel: [w4600 w4605] -> w4591
              frame No Error {
              }
              frame Error {
                n3479 = call <vilib>:"Clear Errors.vi"("error in (no error)"=w4603) -> ("error out"=w4602:errorcluster)  [unwired: 5 in, 1 out]
                n3480 = call "Instrument fgv.vi"("Enum"=T32."ERROR INIT", "error in (no error) 2"=w4602, "INPUT"=w4608) -> ("error"=w4606:errorcluster, "output"=w4607:T18)  [unwired: 6 in, 1 out]
                n3481 = call <vilib>:"Clear Errors.vi"("error in (no error)"=w4606) -> ("error out"=w4605:errorcluster)  [unwired: 5 in, 1 out]
              }
            }
            n3482 = Unbundle By Name(w4590) -> ("LastCom"=→"LastCom UNO":string, "Read Heave and Surge"=→"Read UNO":string)
          }
        }
        n3483 = Unbundle By Name(w4567) -> ("Heave COM Status 2"=w4568:bool, "Heave COM Status"=w4557:bool, "Error Heave"=w4555:errorcluster, "Bytes at Heave Port"=→"Bytes at Humidity Port":dbl)
        n3484 = Not(x=w4557) -> (.not. x?=w4565:bool)
        n3485 = Not(x=w4568) -> (.not. x?=w4556:bool)
        n3486 = local write "Instrument Status"(w4565) -> ()
        n3487 = local write "Error  2"(w4555) -> ()
        n3488 = local write "Port 1a"(w4557) -> ()
        n3489 = local read "Quit"() -> (w4559:bool)
        n3490 = local write "COM Status"(w4556) -> ()
        n3491 = Select(t=enum16{"init", "MAIN", "Panel Close"}."Panel Close", s=w4559, f=enum16{"init", "MAIN", "Panel Close"}."MAIN") -> (s? t:f=w4558:enum16{"init", "MAIN", "Panel Close"})
      }
      frame "Panel Close" {
      }
      frame Default {
      }
    }
  }
